vi "Main.vi"() -> ()   [LabVIEW 2020]
uses:
  System.Windows.Forms
  Global_Variable/Global.vi
  <userlib>/_MGI/Menu Building/MenuTypes/MenuStrip/MGI_MenuStrip.lvclass
  <userlib>/_MGI/Menu Building/MenuItemStatusChange/MGI_MenuItemStatusChange.lvclass
  Libraries/S7/S7.lvlib
panel:
  out "扭矩:":dbl format="%#_3g"
  out "角度: 2":dbl format="%#_4g"
  out "提示信息":string
  out "布尔":bool
  out "工位":enum16{"左工位", "右工位"}(ring)
  out "产品编号":string
  out "T2ROC1+2+3":dbl
  out "T1ROC1+2+3":dbl
  out "PROC_1":dbl
  out "T2ROC3":dbl
  out "T1ROC3":dbl
  out "PROC":i32
  out "T2ROC1+2":i32
  out "T1ROC1+2":i32
  out "T2ROC1":i32
  out "动态标定":T1(xcontrol)
  out "可信度":T1(xcontrol) caption="可信度检测"
  in  "Andon":enum32{"未选择", "缺料报警", "质量报警", "故障报警"}(radio)
  in  "菜单":refnum<k24>(container)
  out "传感器特性":T1(xcontrol)
  out "程序固化":T1(xcontrol)
  out "静态标定":T1(xcontrol)
  in  "Result":string[][](table)
  out "userStatus":string caption="用户状态"
  out "userName":string caption="用户名"
  out "connectionMode":string caption="联机类型"
  out "产品型号":string
  out "PLC":bool
  out "时间字符串":string
  out "日期字符串":string
  out "自动":bool
  out "用时：":u16 format="%#_6u S"
  out "生产数量":i32
  out "合格数量":i32
  out "T1ROC1":i32
  in  "更换产品":refnum<vi>
  out "错误":bool
  # "传感器对中台"
  # "工位一"
  # "检测项目"
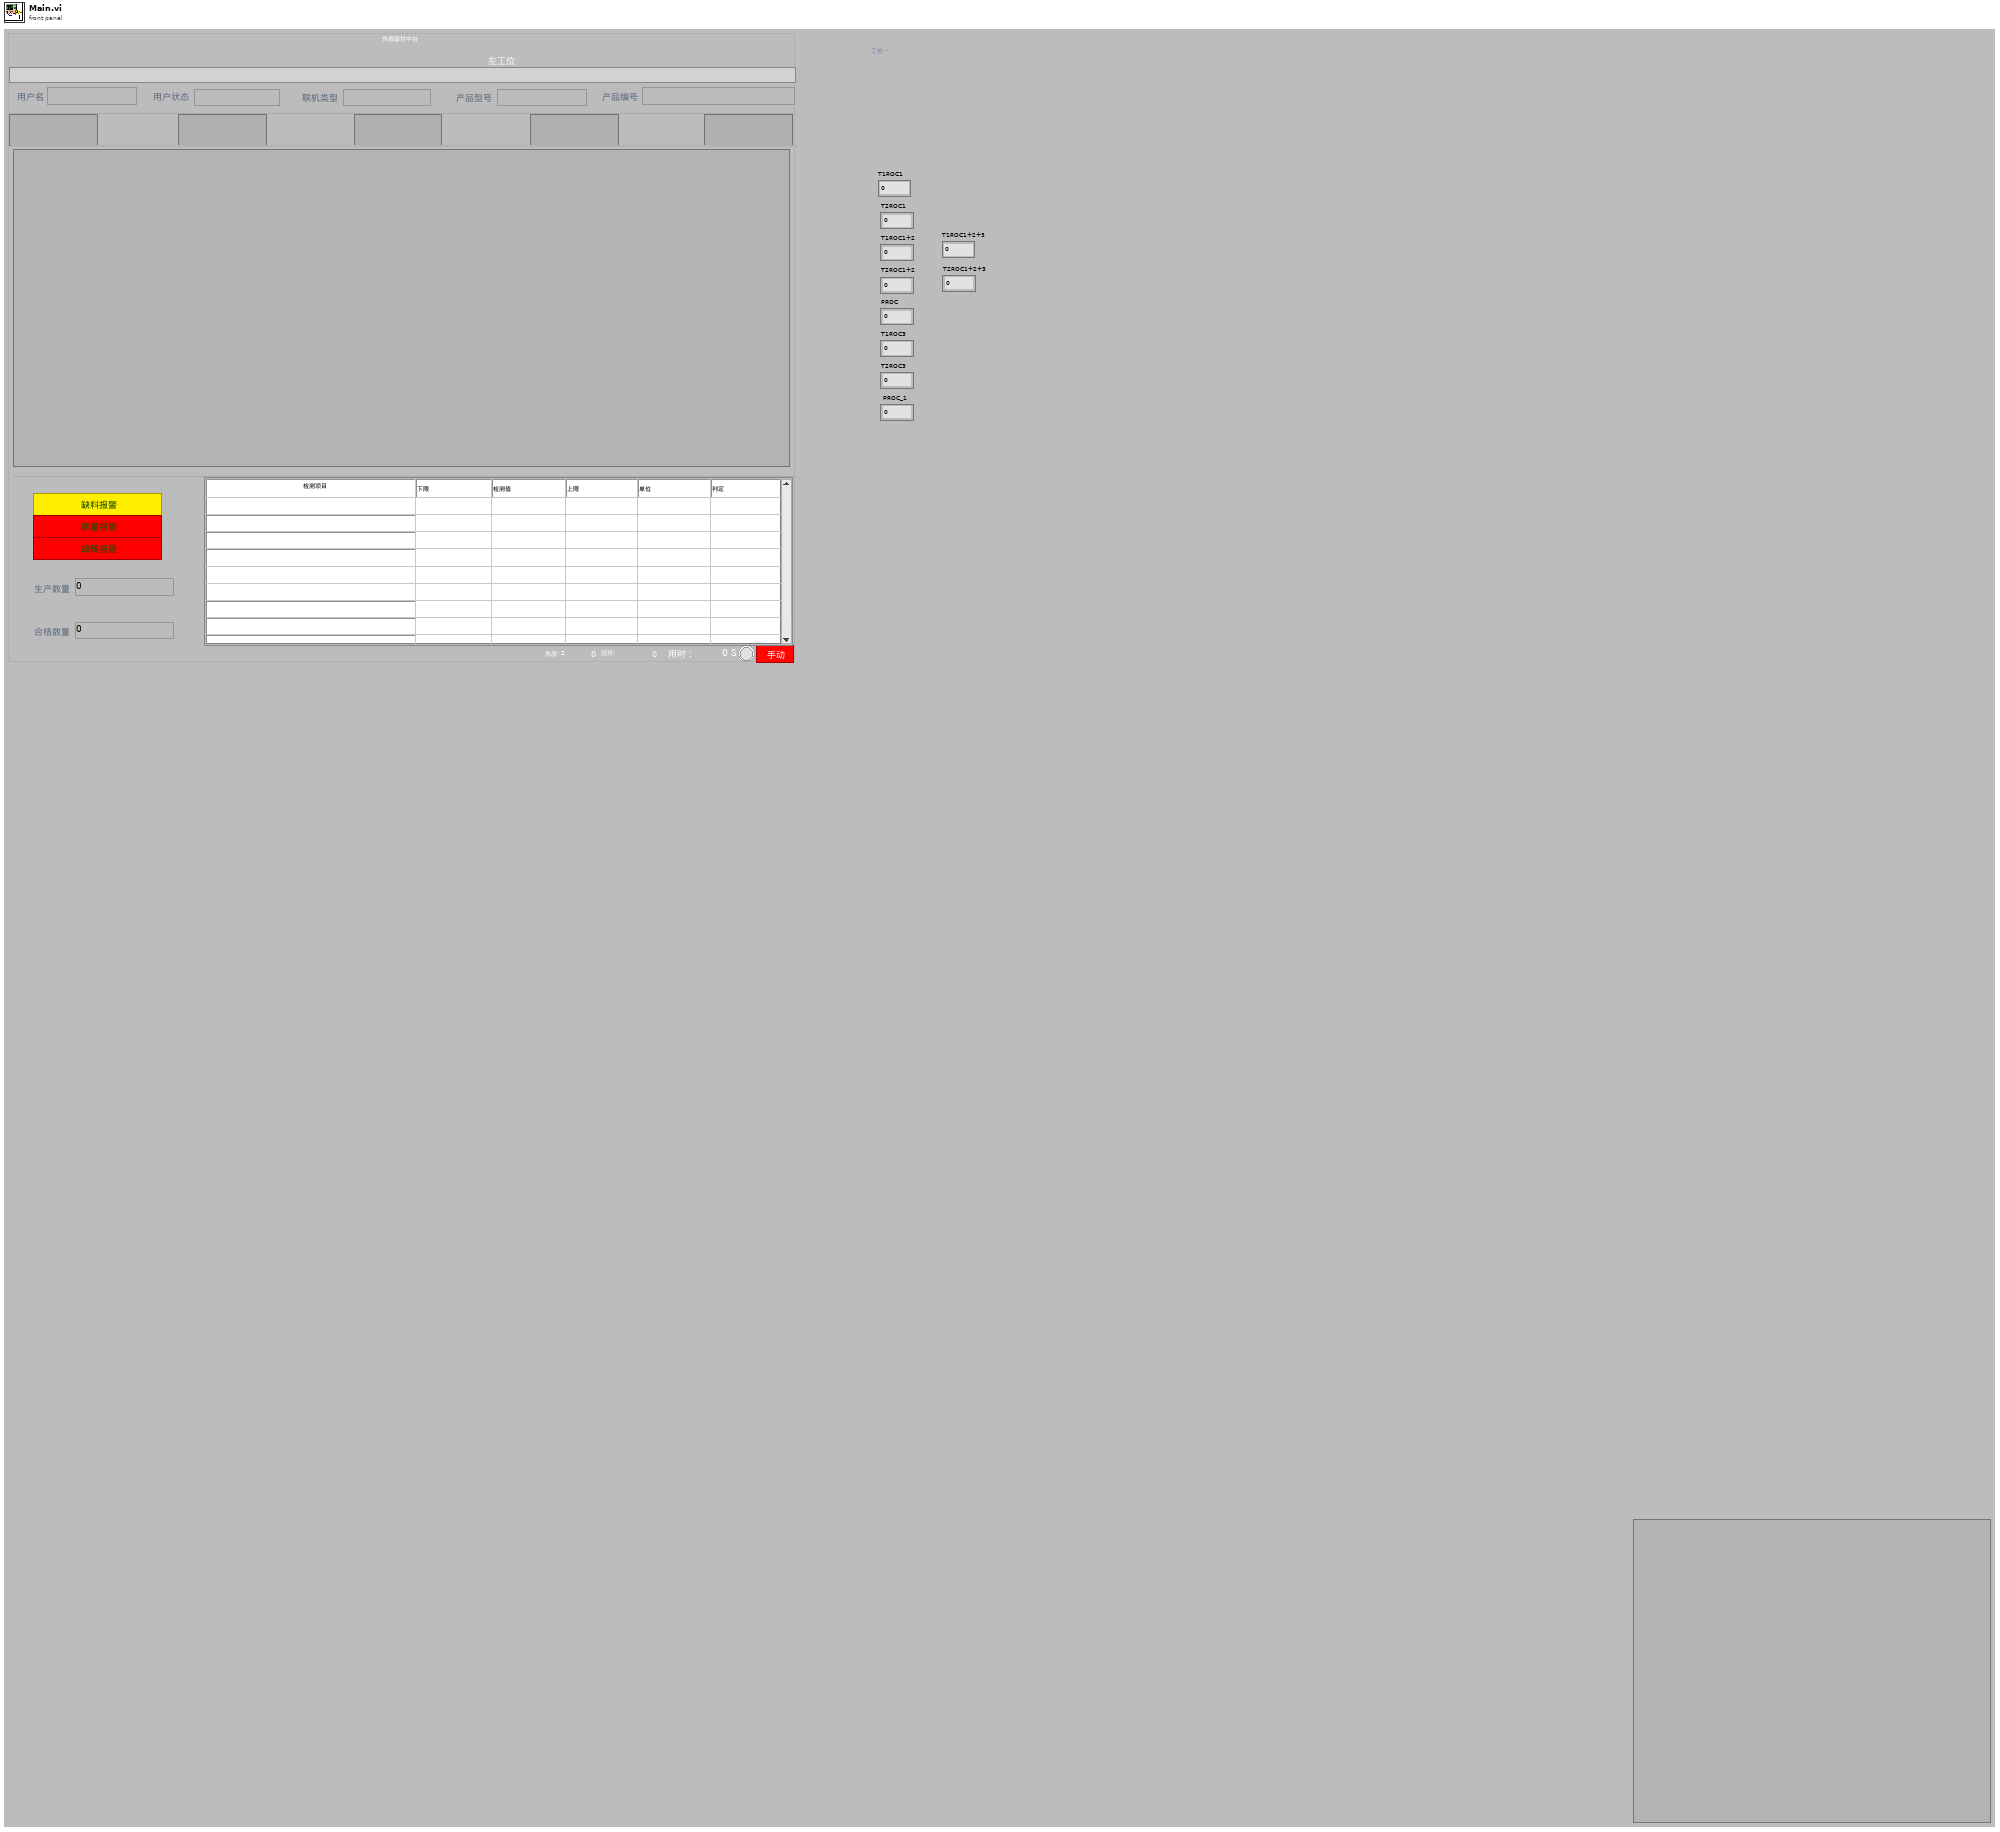
[diagram p1: front panel]
types:
  T1 = enum16{"Idle", "Runing", "Pass", "Faild", "Skip"}
  T2 = typedef "S7.lvlib/Broadcast Events--cluster.ctl" = cluster{"Module Did Init":refnum<user-event>, "Status Updated":refnum<user-event>, "Error Reported":refnum<user-event>, "Module Did Stop":refnum<user-event>, "Update Module Execution Status":refnum<user-event>}
  T3 = cluster{"设备名称":string, "操作人员":string, "设备状态":enum16{"设备离线", "设备正常", "设备缺料", "设备故障", "质量报警"}, "附加信息":string}
  T4 = enum32{"Invalid", "Standard", "Closed", "Hidden", "Minimized", "Maximized"}
  T5 = enum32{"invalid app kind", "Development System", "Run Time System", "Student Edition", "Embedded LabVIEW", "Evaluation", "Custom"}
  T6 = cluster{"工位一驱动伺服位移":sgl, "工位二驱动伺服位移":sgl, "工位一移载伺服位移":sgl, "工位二移载伺服位移":sgl, "工位一编码器位移":sgl, "工位二编码器位移":sgl, "工位一扭矩":sgl, "工位二扭矩":sgl}
  T7 = cluster{"操作员编号":string, "操作员姓名":string, "操作员权限":string, "联机模式":enum16{"单机", "追溯"}}
  T8 = cluster{"Core":cluster{"Current VI Reference":refnum<vi>, "Close Panel on Exit?":bool}, "Your Boolean data":bool, "Your string data":string}
  T9 = cluster{"Current VI Reference":refnum<vi>, "Close Panel on Exit?":bool}
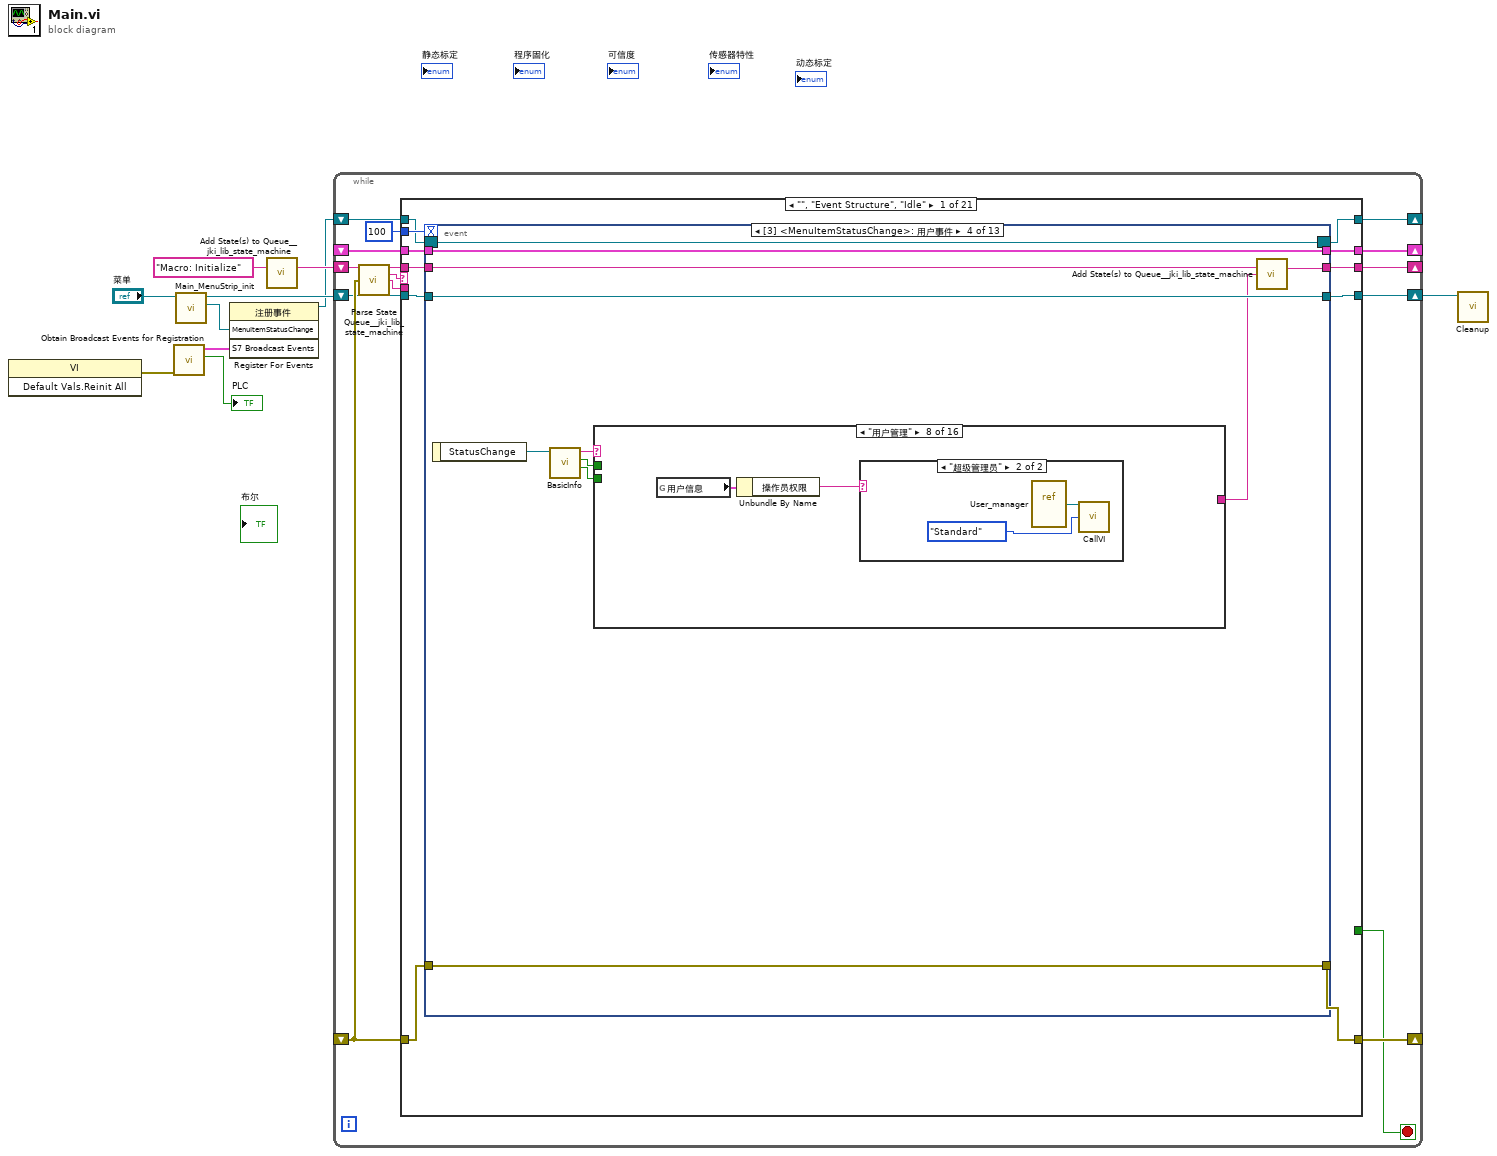
[diagram p0: block diagram]
diagram:
  n1 = invoke class="VI" method="Default Vals.Reinit All"() -> (error out=w3:errorcluster)  [unwired: 3 in, 2 out]
  n2 = call "Obtain Broadcast Events for Registration.vi"("error in (no error)"=w3) -> ("Already running?"=→"PLC":bool, "S7 Broadcast Events"=w5:T2)  [unwired: 8 in, 1 out]
  n3 = call "Main_MenuStrip_init.vi"("MenuStrip"="菜单") -> ("MenuItemStatusChange"=w2:refnum<user-event>, "Menu out"=w7:refnum<class "MGI_MenuStrip.lvclass">)  [unwired: 9 in]
  n4 = register-events(w2, w5) -> (reference out=w1:refnum<event-registration>)  [unwired: 2 in, 1 out]
  n5 = call <vilib>:"Add State(s) to Queue__jki_lib_state_machine.vi"("State(s) in (\"\")"="Macro: Initialize") -> ("States Out"=w10:string)  [unwired: 14 in]
  n6 = while "JKI - String-Based Queued State Machine (Basic) v1.0" {
    shift-right: [w19] -> _
    shift-left: _ -> [w18]
    shift-right: [w21] -> _
    shift-left: _ -> [w16]
    shift-right: [w20] -> _
    shift-left: w10 -> [w22]
    shift-right: [w14] -> w6
    shift-left: w7 -> [w15]
    shift-right: [w12] -> _
    shift-left: w1 -> [w11]
    stop <- w13 stop-if-true
    # "JKI - String-Based Queued State Machine (Basic) v1.0"
    n7 = call <vilib>:"Parse State Queue__jki_lib_state_machine.vi"("State Queue"=w22, "Error In (no error)"=w16) -> ("Remaining States"=w24:string, "Current State"=w25:string, "Arguments"=w23:string)  [unwired: 11 in]
    n8 = case shown="\"\", \"Event Structure\", \"Idle\"" w25 {
      selector: w25 -> [_ _ w283 _ _ _ _ _ _ _ _ _ _ _ _ _ _ _ _ _ _]
      tunnel: w24 -> [w36 w280 w287 w307 w315 w322 w328 w332 w338 w347 w359 w367 w373 w390 w419 w451 w459 w472 w500 w507 w519]
      tunnel: w23 -> [_ _ _ _ _ _ _ _ _ _ _ _ _ _ _ _ w454 w466 _ _ _]
      tunnel: w18 -> [w34 w277 w285 w298 w312 w320 w325 w333 w341 w344 _ w362 w370 w388 w417 w448 w457 w468 w497 w504 w516]
      tunnel: [w33 w278 w289 w304 errorcluster {"status"=FALSE, "code"=0, "source"=""} ("error out") w319 w326 w330 w336 w345 w356 w363 w371 w375 w415 w449 w455 w469 w498 w505 w517] -> w21
      tunnel: w16 -> [w32 w278 w288 w304 w311 w319 w326 w330 w337 w345 w356 w364 w371 w385 w415 w449 w456 w470 w498 w505 w517]
      tunnel: [w35 w279 w286 w306 w314 w321 w327 w332 w339 w346 w358 w366 w372 w389 w418 w450 w458 w471 w499 w506 w518] -> w20
      tunnel: [w31 w277 w285 w305 w312 w320 w325 w333 w341 w344 w357 w362 w370 w388 w417 w448 w457 w468 w497 w504 w516] -> w19
      tunnel: 100 ("Timeout") -> [w30 _ _ _ _ _ _ _ _ _ _ _ _ _ _ _ _ _ _ _ _]
      tunnel: w15 -> [w29 w276 w282 w295 w309 w318 w324 w331 w340 w343 w350 w361 w369 w387 w416 w447 w453 w465 w496 w502 w509]
      tunnel: [w28 w276 w282 w295 w309 w318 w324 w331 w340 w343 w350 w361 w369 w387 w416 w447 w453 w465 w496 w502 w509] -> w14
      tunnel: [_ _ _ _ _ TRUE _ _ _ _ _ _ _ _ _ _ _ _ _ _ _] -> w13
      tunnel: [w26 w275 w281 w294 w308 w316 w323 w334 w335 w342 w351 w360 w368 w386 w414 w446 w452 w464 w495 w501 w508] -> w12
      tunnel: w11 -> [w27 w275 w281 w294 w308 w316 w323 w334 w335 w342 w351 w360 w368 w386 w414 w446 w452 w464 w495 w501 w508]
      frame "", "Event Structure", "Idle" {
        n9 = event shown="[3] <MenuItemStatusChange>: 用户事件" {
          selector: w27 -> [w52 _ w94 w105 w175 w182 w189 w196 w212 w247 w250 w257 w265]
          dyn-events: [w52 _ w93 w105 w175 w182 w189 w196 w212 w247 w250 w257 w265] -> w26
          timeout: w30 -> [_ _ _ _ _ _ _ _ _ _ _ _ _]
          tunnel: w36 -> [w64 w83 w103 w114 w176 w183 w192 w199 w209 w245 w254 w264 w267]
          tunnel: [w63 w83 w103 w112 w177 w184 w193 w200 w210 w244 w255 w263 w268] -> w35
          tunnel: w34 -> [w62 w82 w104 w113 w179 w187 w194 w201 w211 w246 w256 w261 w270]
          tunnel: [w53 w85 w95 w115 w180 w185 w190 w202 w207 w242 w253 w262 w269] -> w33
          tunnel: w32 -> [w53 w85 w96 w115 w180 w185 w190 w203 w207 w242 w253 w262 w269]
          tunnel: [w62 w82 w104 w113 w179 w187 w194 w201 w211 w246 w256 w261 w270] -> w31
          tunnel: w29 -> [w51 w84 w102 w108 w178 w186 w191 w198 w208 w243 _ _ _]
          tunnel: [w51 w84 w102 w108 w178 w186 w191 w198 w208 w243 _ _ _] -> w28
          event Timeout {
            n10 = event-data() -> ()  [unwired: 1 in, 1 out]
            n11 = call "传感器数据.vi"() -> ("传感器读数"=w37:T6)  [unwired: 11 in]
            n12 = global read "Global.vi" "工位"() -> (w39:enum16{"左工位", "右工位"})
            n13 = global read "Global.vi" "扭矩"() -> (w38:cluster{"工位一":dbl, "工位二":dbl})
            n14 = global read "Global.vi" "计时开始"() -> (w55:bool)
            n15 = case shown="\"右工位\"" w39 {
              tunnel: w38 -> [_ _]
              tunnel: w37 -> [w67 w70]
              frame "左工位", Default {
                n16 = Unbundle By Name(w67) -> ("工位一驱动伺服位移"=w66:sgl)
                n17 = global read "Global.vi" "工位一扭矩"() -> (w65:dbl)
                n18 = local write "角度: 2"(w66) -> ()
                n19 = local write "扭矩:"(w65) -> ()
              }
              frame "右工位" {
                n20 = Unbundle By Name(w70) -> ("工位二驱动伺服位移"=w69:sgl)
                n21 = global read "Global.vi" "工位二扭矩"() -> (w68:dbl)
                n22 = local write "角度: 2"(w69) -> ()
                n23 = local write "扭矩:"(w68) -> ()
              }
            }
            n24 = case shown="真" w55 {
              frame False {
                n25 = global write "Global.vi" "计时复位"(TRUE ("计时复位")) -> ()
              }
              frame True {
                n26 = stacked-sequence {
                  frame #0 {
                    n27 = global read "Global.vi" "计时复位"() -> (w72:bool)
                    n28 = call "已用时间"("Reset"=w72) -> ("Elapsed Time (s)"=→"用时：":dbl)  [unwired: 11 in, 7 out]
                  }
                  frame #1 {
                    n29 = global write "Global.vi" "计时复位"(FALSE ("计时复位")) -> ()
                  }
                }
              }
            }
            n30 = Format Date/Time String(time format string (%c)="%H:%M ") -> (date/time string=→"时间字符串":string)  [unwired: 2 in]
            n31 = Format Date/Time String(time format string (%c)="%Y年%m月%d日") -> (date/time string=→"日期字符串":string)  [unwired: 2 in]
            n32 = global read "Global.vi" "T2ROC_1+T2ROC_2"() -> (→"T2ROC1+2":i32)
            n33 = global read "Global.vi" "T1ROC_1+T1ROC_2"() -> (→"T1ROC1+2":i32)
            n34 = global read "Global.vi" "T1ROC_1"() -> (→"T1ROC1":i32)
            n35 = global read "Global.vi" "T2ROC_1"() -> (→"T2ROC1":i32)
            n36 = global read "Global.vi" "PROC"() -> (→"PROC":i32)
            n37 = global read "Global.vi" "产品编号"() -> (→"产品编号":string)
            n38 = global read "Global.vi" "T2ROC1+2+3"() -> (→"T2ROC1+2+3":i32)
            n39 = global read "Global.vi" "T1ROC1+2+3"() -> (→"T1ROC1+2+3":i32)
            n40 = global read "Global.vi" "T1ROC3"() -> (→"T1ROC3":i32)
            n41 = global read "Global.vi" "产品型号"() -> (w40:string)
            n42 = global read "Global.vi" "T2ROC3"() -> (→"T2ROC3":i32)
            n43 = global read "Global.vi" "PROC_1"() -> (→"PROC_1":i32)
            n44 = call <vilib>:"Add State(s) to Queue__jki_lib_state_machine.vi"("State(s) in (\"\")"=w64) -> ("States Out"=w63:string)  [unwired: 14 in]
            n45 = global read "Global.vi" "合格数量"() -> (→"合格数量":i32)
            n46 = global read "Global.vi" "生产数量"() -> (→"生产数量":i32)
            n47 = local write "产品型号"(w40) -> ()
          }
          event "Andon": Value Change {
            w80 = "传感器对中台" ("设备名称")
            n48 = event-data() -> ("NewVal"=w75:enum32{"未选择", "缺料报警", "质量报警", "故障报警"})  [unwired: 1 in]
            n49 = global read "用户信息.vi" "用户信息"() -> (w81:T7)
            n50 = Unbundle By Name(w81) -> ("操作员姓名"=w79:string)
            n51 = case shown="\"故障报警\"" w75 {
              tunnel: w80 -> [_ _ _ _]
              tunnel: w79 -> [_ _ _ _]
              tunnel: [enum16{"设备离线", "设备正常", "设备缺料", "设备故障", "质量报警"}."设备正常" ("设备状态") enum16{"设备离线", "设备正常", "设备缺料", "设备故障", "质量报警"}."设备缺料" ("设备状态") enum16{"设备离线", "设备正常", "设备缺料", "设备故障", "质量报警"}."质量报警" ("设备状态") enum16{"设备离线", "设备正常", "设备缺料", "设备故障", "质量报警"}."设备故障" ("设备状态")] -> w77
              frame "未选择", Default {
              }
              frame "缺料报警" {
              }
              frame "质量报警" {
              }
              frame "故障报警" {
              }
            }
            n52 = Bundle By Name(cluster=T3 {"设备名称"="", "操作人员"="", "设备状态"=enum."设备离线", "附加信息"=""} ("设备信息"), "设备名称"=w80, "操作人员"=w79, "设备状态"=w77) -> (w76:T3)
            n53 = call "Change_Client.vi"("设备信息"=w76) -> ()  [unwired: 10 in, 1 out]
          }
          event "PLC": Value Change; "PLC": Mouse Down {
            n54 = event-data() -> ()  [unwired: 1 in, 4 out]
            n55 = call "Start Module.vi"("error in (no error)"=w96) -> ("error out"=w92:errorcluster, "Wait for Event Sync?"=w101:bool, "S7 Broadcast Events"=w100:T2, "Module Was Already Running?"=w99:bool)  [unwired: 7 in]
            n56 = local write "PLC"(w99) -> ()
            n57 = register-events(reference=w94, error in=w92, w100) -> (reference out=w93:refnum<event-registration>, error out=w91:errorcluster)  [unwired: 1 in]
            n58 = call "Synchronize Module Events.vi"("error in (no error)"=w91, "Wait for Event Sync?"=w101) -> ("error out"=w90:errorcluster)  [unwired: 9 in]
            n59 = call "Init S7 Link.vi"("error in (no error)"=w90, "超时"=500, "IP"="192.168.0.11") -> ("error out"=w95:errorcluster)  [unwired: 8 in]
          }
          event User Event {
            n60 = event-data() -> ("StatusChange"=w106:refnum<class "MGI_MenuItemStatusChange.lvclass">)  [unwired: 1 in]
            n61 = call <userlib>:"BasicInfo.vi"("MGI_MenuItemStatusChange in"=w106) -> ("Enabled?"=w109:bool, "Checked?"=w110:bool, "Tag"=w111:string)  [unwired: 7 in, 1 out]
            n62 = case shown="\"用户管理\"" w111 {
              tunnel: w110 -> [_ _ _ _ _ _ _ _ _ _ _ _ _ _ _ _]
              tunnel: w109 -> [_ _ _ _ _ _ _ _ _ _ _ _ _ _ _ _]
              tunnel: [_ _ "S7: Stop\nMacro: Exit" _ _ _ _ _ _ _ _ _ _ _ _ _] -> w107
              frame "假", Default {
              }
              frame "数据库配置" {
                n63 = global read "用户信息.vi" "用户信息"() -> (w117:T7)
                n64 = Unbundle By Name(w117) -> ("操作员权限"=w116:string)
                n65 = case shown="\"超级管理员\", \"系统管理员\"" w116 {
                  frame Default {
                    n66 = One Button Dialog(message="权限不足！" ("消息")) -> ()  [unwired: 1 in, 1 out]
                  }
                  frame "超级管理员", "系统管理员" {
                    n67 = vi-ref "数据库配置.vi"() -> (w120:refnum<vi>)
                    n68 = call "CallVI.vi"("VI引用"=w120, "状态"=T4."Standard") -> ()  [unwired: 12 in, 2 out]
                  }
                }
              }
              frame "退出" {
                n69 = call "Close_Client.vi"() -> ()  [unwired: 12 in]
              }
              frame "手动控制" {
                n70 = global read "用户信息.vi" "用户信息"() -> (w123:T7)
                n71 = Unbundle By Name(w123) -> ("操作员权限"=w122:string)
                n72 = case shown="\"班组长\", \"系统管理员\"" w122 {
                  frame Default {
                    n73 = One Button Dialog(message="权限不足！" ("消息")) -> ()  [unwired: 1 in, 1 out]
                  }
                  frame "班组长", "系统管理员" {
                    n74 = vi-ref "IO.vi"() -> (w126:refnum<vi>)
                    n75 = call "CallVI.vi"("VI引用"=w126, "状态"=T4."Standard") -> ()  [unwired: 12 in, 2 out]
                  }
                }
              }
              frame "半自动控制" {
                n76 = disable-structure shown="启用" {
                  frame Disabled {
                    n77 = shared-variable "我的电脑\\Global.lvlib\\操作者权限"() -> (w127:string)  [unwired: 1 in, 1 out]
                    n78 = case shown="\"班组长\", \"系统管理员\"" w127 {
                      frame Default {
                        n79 = One Button Dialog(message="权限不足！" ("消息")) -> ()  [unwired: 1 in, 1 out]
                      }
                      frame "班组长", "系统管理员" {
                        n80 = call "CallVI.vi"("VI引用"=refnum<vi> refnum, "状态"=T4."Maximized") -> ()  [unwired: 12 in, 2 out]
                      }
                    }
                  }
                  frame Enabled {
                    n81 = One Button Dialog(message="当前设备不具备半自动功能！" ("消息")) -> ()  [unwired: 1 in, 1 out]
                  }
                }
              }
              frame "产品管理" {
                n82 = vi-ref "Config.vi"() -> (w133:refnum<vi>)
                n83 = call "CallVI.vi"("VI引用"=w133, "状态"=T4."Standard") -> ()  [unwired: 12 in, 2 out]
              }
              frame "系统配置" {
                n84 = global read "用户信息.vi" "用户信息"() -> (w135:T7)
                n85 = Unbundle By Name(w135) -> ("操作员权限"=w134:string)
                n86 = case shown="\"班组长\", \"超级管理员\", \"系统管理员\"" w134 {
                  frame Default {
                    n87 = One Button Dialog(message="权限不足！" ("消息")) -> ()  [unwired: 1 in, 1 out]
                  }
                  frame "班组长", "超级管理员", "系统管理员" {
                    n88 = vi-ref "Setting.vi"() -> (w138:refnum<vi>)
                    n89 = call "CallVI.vi"("VI引用"=w138, "状态"=T4."Standard") -> ()  [unwired: 12 in, 2 out]
                  }
                }
              }
              frame "用户管理" {
                n90 = global read "用户信息.vi" "用户信息"() -> (w140:T7)
                n91 = Unbundle By Name(w140) -> ("操作员权限"=w139:string)
                n92 = case shown="\"超级管理员\"" w139 {
                  frame Default {
                    n93 = One Button Dialog(message="权限不足！" ("消息")) -> ()  [unwired: 1 in, 1 out]
                  }
                  frame "超级管理员" {
                    n94 = vi-ref "User_manager.vi"() -> (w143:refnum<vi>)
                    n95 = call "CallVI.vi"("VI引用"=w143, "状态"=T4."Standard") -> ()  [unwired: 12 in, 2 out]
                  }
                }
              }
              frame "设备管理" {
                n96 = global read "用户信息.vi" "用户信息"() -> (w145:T7)
                n97 = Unbundle By Name(w145) -> ("操作员权限"=w144:string)
                n98 = case shown="\"超级管理员\", \"系统管理员\"" w144 {
                  frame Default {
                    n99 = One Button Dialog(message="权限不足！" ("消息")) -> ()  [unwired: 1 in, 1 out]
                  }
                  frame "超级管理员", "系统管理员" {
                    n100 = vi-ref "注册设备.vi"() -> (w148:refnum<vi>)
                    n101 = call "CallVI.vi"("VI引用"=w148, "状态"=T4."Standard") -> ()  [unwired: 12 in, 2 out]
                  }
                }
              }
              frame "编码规则" {
                n102 = global read "用户信息.vi" "用户信息"() -> (w150:T7)
                n103 = Unbundle By Name(w150) -> ("操作员权限"=w149:string)
                n104 = case shown="\"班组长\", \"超级管理员\", \"工艺管理员\", \"系统管理员\"" w149 {
                  frame Default {
                    n105 = One Button Dialog(message="权限不足！" ("消息")) -> ()  [unwired: 1 in, 1 out]
                  }
                  frame "班组长", "超级管理员", "工艺管理员", "系统管理员" {
                    n106 = vi-ref "编码规则设置.vi"() -> (w153:refnum<vi>)
                    n107 = call "CallVI.vi"("VI引用"=w153, "状态"=T4."Standard") -> ()  [unwired: 12 in, 2 out]
                  }
                }
              }
              frame "易损件管理" {
                n108 = vi-ref "易损件管理.vi"() -> (w155:refnum<vi>)
                n109 = call "CallVI.vi"("VI引用"=w155, "状态"=T4."Standard") -> ()  [unwired: 12 in, 2 out]
              }
              frame "物料批次管理" {
                n110 = vi-ref "批次管理.vi"() -> (w157:refnum<vi>)
                n111 = call "CallVI.vi"("VI引用"=w157, "状态"=T4."Standard") -> ()  [unwired: 12 in, 2 out]
              }
              frame "报表" {
                n112 = call "文件对话框"("start path"=path "D:/report", "prompt"="打开报表", "pattern (all files)"="*.doc;*.docx", "pattern label"="Word 文档") -> ("selected path"=w158:path, "error out"=w159:errorcluster)  [unwired: 8 in, 2 out]
                n113 = case shown="无错误" w159 {
                  selector: w159 -> [w165 w167]
                  tunnel: w158 -> [w166 _]
                  frame No Error {
                    w164 = 1 items=["Normal", "Maximize", "Minimize"] ("cpubbs_WindowState")
                    n114 = call "Open_Word.vi"("File Path"=w166, "cpubbs_WindowState"=w164, "错误输入（无错误）"=w165) -> ()  [unwired: 12 in, 1 out]
                  }
                  frame Error {
                    n115 = call <vilib>:"Clear Errors.vi"("error in (no error)"=w167) -> ()  [unwired: 5 in, 2 out]
                  }
                }
              }
              frame "报警信息" {
                n116 = vi-ref "报警信息.vi"() -> (w169:refnum<vi>)
                n117 = call "CallVI.vi"("VI引用"=w169, "状态"=T4."Standard") -> ()  [unwired: 12 in, 2 out]
              }
              frame "关于" {
                n118 = vi-ref "About.vi"() -> (w171:refnum<vi>)
                n119 = call "CallVI.vi"("VI引用"=w171, "状态"=T4."Standard") -> ()  [unwired: 12 in, 2 out]
              }
              frame "操作演示" {
                n120 = call <vilib>:"Application Directory.vi"() -> ("Application Directory"=w174:path)
                n121 = Build Path(base path=w174, name or relative path="操作演示" ("名称或相对路径")) -> (appended path=w173:path)
                n122 = call "自动播放ppt.vi"("路径"=w173) -> ()  [unwired: 10 in, 1 out]
              }